vi "UHR-Fleezers Control (host) - 12.7d.vi"() -> ()   [LabVIEW 2012] (continued)
          }
          frame True {
            w4347 = TRUE ("AI to FIFO")
            n2449 = local read "Scan steps (MCL)"() -> (w4326:u64)
            n2450 = local read "Scan lines (y)"() -> (w4322:u64)
            n2451 = local read "Fast Scan Dir"() -> (w4333:bool)
            n2452 = local read "Actual MCL Inc (V)"() -> (w4323:dbl)
            n2453 = Decrement(x=w4322) -> (x-1=w4321:u64)
            n2454 = Decrement(x=w4326) -> (x-1=w4325:u64)
            n2455 = Multiply(x=w4323, y=w4321) -> (x*y=w4320:dbl)
            n2456 = Divide(x=w4320, y=2.0) -> (x/y=w4330:dbl)
            n2457 = Multiply(x=w4323, y=w4325) -> (x*y=w4324:dbl)
            n2458 = Divide(x=w4324, y=2.0) -> (x/y=w4329:dbl)
            n2459 = Select(t=w4329, s=w4333, f=w4330) -> (s? t:f=w4328:dbl)
            n2460 = Select(t=w4330, s=w4333, f=w4329) -> (s? t:f=w4332:dbl)
            n2461 = Subtract(x=w4340, y=w4332) -> (x-y=w4331:dbl)
            n2462 = Subtract(x=w4343, y=w4328) -> (x-y=w4327:dbl)
            n2463 = local read "2D or 1D Scan"() -> (w4345:bool)
            n2464 = Not(x=w4333) -> (.not. x?=w4339:bool)
            n2465 = Not(x=w4345) -> (.not. x?=w4341:bool)
            n2466 = And(x=w4333, y=w4341) -> (x .and. y?=w4342:bool)
            n2467 = And(x=w4341, y=w4339) -> (x .and. y?=w4344:bool)
            n2468 = Select(t=w4343, s=w4344, f=w4327) -> (s? t:f=w4334:dbl)
            n2469 = Select(t=w4340, s=w4342, f=w4331) -> (s? t:f=w4335:dbl)
            n2470 = call "Volt to I16.vi"("Voltage In"=w4335) -> ("I16 Voltage Out"=w4338:i16)
            n2471 = call "Volt to I16.vi"("Voltage In"=w4334) -> ("I16 Voltage Out"=w4337:i16)
            n2472 = xnode "Read/Write Control"("FPGA VI Reference In"=w4351, "error in"=w4350, "AI to FIFO"=w4347, "APD to FIFO"=w4347, "Start scan (MCL)"=w4347, "AO1"=w4338, "AO2"=w4337) -> ("FPGA VI Reference Out"=w4349:T20, "error out"=w4348:errorcluster)
          }
        }
        "Initial Y" <- w4300
        "Initial X" <- w4299
        n2473 = local write "Tab Control 6"(T3."Imaging" ("Tab Control 6")) -> ()
        "wait to reset values" <- w4301
      }
    }
    n2474 = local read "APD Elements/DMA read"() -> (w3455:u32)
    n2475 = local read "Trap AI Elements/DMA read"() -> (w3675:u32)
    n2476 = xnode "Get APD Data"("FPGA VI Reference In"=w3614, "error in"=w3613, "Number of Elements"=w3455, "Timeout (ms)"=-1) -> ("Data"=w3644:u32[], "Elements Remaining"=→"APD FIFO Elements Remaining":u32)  [unwired: 2 out]
    n2477 = local read "Trap Pos Elements/DMA read"() -> (w3610:u32)
    n2478 = xnode "Invoke Method"("FPGA VI Reference In"=w3614, "error in"=w3613, "Number of Elements"=w3610, "Timeout (ms)"=-1) -> ("Data"=w3574:u16[], "Elements Remaining"=→"Trap Pos FIFO El Remaining":u32)  [unwired: 2 out]
    n2479 = xnode "Get Trap Data"("FPGA VI Reference In"=w3614, "error in"=w3613, "Number of Elements"=w3675, "Timeout (ms)"=-1 ("Timeout")) -> ("FPGA VI Reference Out"=w3509:T20, "error out"=w3508:errorcluster, "Data"=w3575:i16[], "Elements Remaining"=w3797:u32)
    "FIFO El. Rem." <- w3797
    n2480 = local read "DMA Update Period (s)"() -> (w3676:dbl)
    n2481 = local read "Trap AI FIFO Depth"() -> (w3799:u32)
    n2482 = local read "Number of APDs"() -> (w3477:u8)
    n2483 = Decimate 1D Array(w3574) -> (w3571:u16[], w3573:u16[], w3572:u16[])
    n2484 = feedback #6(0.0) -> (w3603:dbl)
    n2485 = Add(x=w3676, y=w3603) -> (x+y=w3773:dbl)
    n2486 = feedback-in #6(w3773) -> ()
    n2487 = To Time Stamp(1:w3603) -> (0:w3602:timestamp)
    n2488 = Subtract(x=w3799, y=w3675) -> (x-y=w3798:u32)
    n2489 = To Unsigned Long Integer(number=w3571) -> (unsigned 32bit integer=w3570:u32[])
    n2490 = Join Numbers(hi=w3573, lo=w3572) -> ((hi.lo)=w3569:u32[])
    n2491 = Divide(x=w3797, y=w3798) -> (x/y=w3796:dbl)
    "Buffer Status" <- w3796
    n2492 = case "Deinterlace APD signals" shown="3, Default" w3477 {
      tunnel: [w3809 w3815] -> w3454
      tunnel: w3644 -> [w3810 w3814]
      tunnel: [w3808 w3813] -> w3453
      tunnel: [w3807 w3811] -> w3460
      frame 3, Default {
        n2493 = Decimate 1D Array "APD signals"(w3810) -> (w3809:u32[], w3808:u32[], w3807:u32[])
      }
      frame 2 {
        n2494 = Decimate 1D Array "APD signals"(w3814) -> (w3815:u32[], w3813:u32[])
        n2495 = Multiply(x=w3813, y=u32 0) -> (x*y=w3811:u32[])
      }
    }
    n2496 = Join Numbers(hi=w3570, lo=w3569) -> ((hi.lo)=w3563:u64[])
    n2497 = call "IR AOM word to freq - vec.vi"("Frequency Word In (double vec)"=w3563) -> ("Frequency Out"=w3609:dbl[])
    n2498 = Equal?(x=w3796, y=1.0) -> (x = y?=w3794:bool)
    n2499 = case "Alert buffer overflow" shown="True" w3794 {
      frame False {
      }
      frame True {
        n2500 = call <vilib>:"Beep.vi"() -> ()  [unwired: 3 in, 9 out]
        "Overflow (data lost)" <- TRUE ("Overflow (data lost)")
      }
    }
    n2501 = Decimate 1D Array(w3609) -> (w3608:dbl[], w3607:dbl[])
    n2502 = Build Array(w3608, w3607) -> (w3606:dbl[][])
    n2503 = Bundle(w3454, w3453, w3460) -> (w3458:cluster{u32[], u32[], u32[]})  [unwired: 1 in]
    n2504 = Build Array(w3454, w3453, w3460) -> (w3734:u32[][])
    n2505 = for {
      tunnel: w3454 -> [w3805] mode=indexing
      n2506 = call "Smart Buffer (DBL) 1.vi"("new element [write]"=w3805, "mode"=T21."write") -> ()  [unwired: 4 in, 6 out]
    }
    n2507 = local read "APD Integration Time (s)"() -> (w3470:dbl)
    n2508 = To Double Precision Float(number=w3734) -> (double precision float=w3735:dbl[][])
    n2509 = feedback #7 "APD3"(w3460) -> (w3476:u32[])
    n2510 = feedback #8 "APD2"(w3453) -> (w3632:u32[])
    n2511 = feedback #9 "APD1"(w3454) -> (w3733:u32[])
    n2512 = Build Array (concatenate)(w3632, w3453) -> (w3631:u32[])
    n2513 = Build Array (concatenate)(w3476, w3460) -> (w3475:u32[])
    n2514 = Build Array (concatenate)(w3733, w3454) -> (w3730:u32[])
    n2515 = for {
      tunnel: w3453 -> [w3804] mode=indexing
      n2516 = call "Smart Buffer (DBL) 2.vi"("new element [write]"=w3804, "mode"=T21."write") -> ()  [unwired: 4 in, 6 out]
    }
    n2517 = Array Size(array=w3730) -> (size(s)=w3727:i32)
    n2518 = Array Size(array=w3454) -> (size(s)=w3729:i32)
    n2519 = Multiply(x=w3729, y="APD Ave N") -> (x*y=w3728:dbl)
    n2520 = Greater?(x=w3727, y=w3728) -> (0:w3731:bool)
    n2521 = Bundle("APD 1", "APD 2", "APD 3") -> (w3767:cluster{string, string, string})  [unwired: 1 out]
    n2522 = local read "Trap Sets"() -> (w3674:u32)
    n2523 = case shown="True" w3731 {
      tunnel: w3730 -> [w4107 w4116]
      tunnel: [w4107 w4114] -> w3681
      tunnel: w3728 -> [_ w4109]
      tunnel: w3727 -> [_ w4115]
      tunnel: w3631 -> [w4106 w4113]
      tunnel: [w4106 w4112] -> w3629
      tunnel: w3475 -> [w4105 w4111]
      tunnel: [w4105 w4108] -> w3471
      frame False {
      }
      frame True {
        n2524 = Subtract(x=w4115, y=w4109) -> (x-y=w4110:dbl)
        n2525 = Array Subset "APD3"(array=w4111, index=w4110, length=w4109) -> (w4108:u32[])
        n2526 = Array Subset "APD2"(array=w4113, index=w4110, length=w4109) -> (w4112:u32[])
        n2527 = Array Subset "APD1"(array=w4116, index=w4110, length=w4109) -> (w4114:u32[])
      }
    }
    n2528 = feedback-in #7(w3471) -> ()
    n2529 = feedback-in #8(w3629) -> ()
    n2530 = feedback-in #9(w3681) -> ()
    n2531 = Cluster To Array(cluster=w3767) -> (array=w3764:string[])
    n2532 = for "APD" {
      tunnel: w3735 -> [w4363] mode=indexing
      tunnel: w3470 -> [w4370]
      tunnel: [w4366] -> w3633 mode=indexing
      tunnel: "APD Disp. Scale" -> [w4367]
      tunnel: w3764 -> [w4365] mode=indexing
      tunnel: "APD Disp. Downsample" -> [w4361]
      tunnel: [w4364] -> w3763
      workers-P: _ -> [_]
      tunnel: w3602 -> [w4360]
      n2533 = call "integrate 1D array interval - double.vi"("Ave N"=w4361, "Array In"=w4363) -> ("Array Out"=w4362:dbl[])  [unwired: 1 out]
      n2534 = Multiply(x=w4370, y=w4361) -> (x*y=w4364:dbl)
      n2535 = Divide(x=w4362, y=w4367) -> (x/y=w4368:dbl[])
      n2536 = Bundle By Name("t0"=w4360, "Y"=w4368, "dt"=w4364) -> (w4369:waveform(dbl))  [unwired: 1 out]
      n2537 = Set Waveform Attribute(5:w4365, 6:"NI_ChannelName" ("name"), 7:w4369) -> (3:w4366:waveform(dbl))  [unwired: 1 in, 2 out]
    }
    "APD Display Period (s)" <- w3763
    n2538 = Reciprocal(x=w3763) -> (1/x=→"APD Display Freq. (Hz)":dbl)
    n2539 = case "Deinterlace trap data, average down PSD" shown="2" w3674 {
      tunnel: w3575 -> [w4388 w4453]
      tunnel: [w4385 w4450] -> w3667
      tunnel: [w4388 w4452] -> w3566
      tunnel: "Detector Type" -> [w4387 w4448]
      tunnel: [w4386 w4451] -> w3666
      tunnel: [w4384 w4449] -> w3771
      frame 1, Default {
        n2540 = Divide(x=w4388, y=3276.7) -> (x/y=w4389:dbl[])
        n2541 = Decimate 1D Array(w4389) -> (w4398:dbl[], w4397:dbl[], w4396:dbl[], w4395:dbl[], w4394:dbl[], w4393:dbl[], w4392:dbl[], w4391:dbl[])
        n2542 = case shown="\"IR-QPD + PSD + FB-QPD position\"" w4387 {
          tunnel: w4398 -> [w4422 w4447]
          tunnel: w4397 -> [w4421 w4446]
          tunnel: w4396 -> [w4406 w4424]
          tunnel: w4395 -> [w4407 w4434]
          tunnel: w4394 -> [w4420 w4445]
          tunnel: w4393 -> [w4419 w4444]
          tunnel: w4392 -> [w4403 w4425]
          tunnel: w4391 -> [w4402 w4423]
          tunnel: [w4401 w4431] -> w4386
          tunnel: [w4400 w4430] -> w4385
          tunnel: [w4399 w4429] -> w4384
          frame "IR-QPD + PSD + FB-QPD", Default {
            w4399 = 0  # Channel pattern
            n2543 = Divide(x=w4422, y=w4407) -> (x/y=w4409:dbl[])
            n2544 = Divide(x=w4421, y=w4407) -> (x/y=w4408:dbl[])
            n2545 = Divide(x=w4420, y=w4403) -> (x/y=w4405:dbl[])
            n2546 = Divide(x=w4419, y=w4402) -> (x/y=w4404:dbl[])
            n2547 = Build Array(w4409, w4408, w4407, w4406, w4405, w4404, w4403, w4402) -> (w4400:dbl[][])
            n2548 = Bundle("T1 Y", "T1 X", "T1 Sum", "FB Sum", "PSD Y", "PSD X", "PSD Y Sum", "PSD X Sum") -> (w4418:T44)  [unwired: 1 out]
            n2549 = Cluster To Array(cluster=w4418) -> (array=w4401:string[])
          }
          frame "IR-QPD + PSD + FB-QPD position" {
            w4429 = 3  # Channel pattern
            n2550 = Negate(x=w4425) -> (-x=w4426:dbl[])
            n2551 = Divide(x=w4447, y=w4434) -> (x/y=w4436:dbl[])
            n2552 = Divide(x=w4446, y=w4434) -> (x/y=w4435:dbl[])
            n2553 = Divide(x=w4445, y=w4425) -> (x/y=w4433:dbl[])
            n2554 = Divide(x=w4444, y=w4426) -> (x/y=w4432:dbl[])
            n2555 = Build Array(w4436, w4435, w4434, w4423, w4424, w4433, w4432, w4425) -> (w4430:dbl[][])
            n2556 = Bundle("T1 Y", "T1 X", "T1 Sum", "FB X", "FB Sum", "PSD Y", "PSD X", "PSD Y Sum") -> (w4443:T44)  [unwired: 1 out]
            n2557 = Cluster To Array(cluster=w4443) -> (array=w4431:string[])
          }
        }
      }
      frame 2 {
        n2558 = case shown="\"IR-QPD + PSD + FB-QPD X position\"" w4448 {
          tunnel: w4453 -> [w4515 w4587 w4658]
          tunnel: [w4454 w4578 w4589] -> w4452
          tunnel: [w4481 w4569 w4636] -> w4451
          tunnel: [w4480 w4532 w4603] -> w4450
          tunnel: [w4474 w4567 w4634] -> w4449
          frame "IR-QPD + PSD + FB-QPD", Default {
            w4474 = 1  # Channel pattern
            # "time average x2 the 4th signal and the 4 psd signals (detection laser)"
            # "deinterlace 3 signals from qpd"
            n2559 = Decimate 1D Array(w4515) -> (w4514:i16[], w4513:i16[], w4479:i16[], w4512:i16[], w4502:i16[], w4500:i16[], w4499:i16[], w4497:i16[])
            n2560 = Decimate 1D Array(w4479) -> (w4478:i16[], w4477:i16[])
            n2561 = Decimate 1D Array(w4514) -> (w4511:i16[], w4483:i16[])
            n2562 = Decimate 1D Array(w4513) -> (w4510:i16[], w4508:i16[])
            n2563 = Decimate 1D Array(w4512) -> (w4509:i16[], w4507:i16[])
            n2564 = call "downsample 1D array - double.vi"("Ave N"=2.0, "Array In"=w4502) -> ("Array Out"=w4501:dbl[])  [unwired: 1 out]
            n2565 = call "downsample 1D array - double.vi"("Ave N"=2.0, "Array In"=w4500) -> ("Array Out"=w4482:dbl[])  [unwired: 1 out]
            n2566 = call "downsample 1D array - double.vi"("Ave N"=2.0, "Array In"=w4499) -> ("Array Out"=w4498:dbl[])  [unwired: 1 out]
            n2567 = call "downsample 1D array - double.vi"("Ave N"=2.0, "Array In"=w4497) -> ("Array Out"=w4496:dbl[])  [unwired: 1 out]
            n2568 = Interleave 1D Arrays(w4511, w4510, w4509, w4483, w4508, w4507, w4478, w4477, w4501, w4482, w4498, w4496) -> (w4495:dbl[])
            n2569 = Divide(x=w4495, y=3276.7) -> (x/y=w4494:dbl[])
            n2570 = Decimate 1D Array(w4494) -> (w4493:dbl[], w4492:dbl[], w4491:dbl[], w4490:dbl[], w4489:dbl[], w4488:dbl[], w4476:dbl[], w4475:dbl[], w4487:dbl[], w4486:dbl[], w4485:dbl[], w4484:dbl[])
            n2571 = Divide(x=w4493, y=w4491) -> (x/y=w4461:dbl[])
            n2572 = Divide(x=w4492, y=w4491) -> (x/y=w4460:dbl[])
            n2573 = Divide(x=w4490, y=w4488) -> (x/y=w4459:dbl[])
            n2574 = Divide(x=w4489, y=w4488) -> (x/y=w4458:dbl[])
            n2575 = Divide(x=w4487, y=w4485) -> (x/y=w4457:dbl[])
            n2576 = Divide(x=w4486, y=w4484) -> (x/y=w4456:dbl[])
            n2577 = Build Array(w4461, w4460, w4491, w4459, w4458, w4488, w4476, w4475, w4457, w4456, w4485, w4484) -> (w4480:dbl[][])
            n2578 = Bundle("T1 Y", "T1 X", "T1 Sum", "T2 Y", "T2 X", "T2 Sum", "T1 FB Sum", "T2 FB Sum", "PSD Y", "PSD X", "PSD Y Sum", "PSD X Sum") -> (w4462:T45)  [unwired: 1 out]
            n2579 = To Word Integer(number=w4495) -> (16bit integer=w4454:i16[])
            n2580 = Cluster To Array(cluster=w4462) -> (array=w4481:string[])
          }
          frame "IR-QPD + PSD + FB-QPD X position" {
            w4567 = 2  # Channel pattern
            # "time average x2 the 3 psd signals (detection laser)"
            # "deinterlace 3 signals from qpds"
            n2581 = Decimate 1D Array(w4587) -> (w4586:i16[], w4585:i16[], w4568:i16[], w4584:i16[], w4530:i16[], w4527:i16[], w4524:i16[], w4555:i16[])
            n2582 = Select(t=i16 -1, s="Flip X Sign", f=i16 1) -> (s? t:f=w4520:i16)
            n2583 = Multiply(x=w4585, y=w4520) -> (x*y=w4521:i16[])
            n2584 = Decimate 1D Array(w4568) -> (w4553:i16[], w4551:i16[])
            n2585 = Decimate 1D Array(w4586) -> (w4583:i16[], w4570:i16[])
            n2586 = Decimate 1D Array(w4521) -> (w4582:i16[], w4580:i16[])
            n2587 = Decimate 1D Array(w4584) -> (w4581:i16[], w4579:i16[])
            n2588 = Decimate 1D Array(w4555) -> (w4554:i16[], w4552:i16[])
            n2589 = call "downsample 1D array - I16.vi"("Ave N"=2.0, "Array In"=w4530) -> ("Array Out"=w4528:i16[])  [unwired: 1 in]
            n2590 = call "downsample 1D array - I16.vi"("Ave N"=2.0, "Array In"=w4524) -> ("Array Out"=w4522:i16[])  [unwired: 1 in]
            n2591 = call "downsample 1D array - I16.vi"("Ave N"=2.0, "Array In"=w4527) -> ("Array Out"=w4525:i16[])  [unwired: 1 in]
            n2592 = Interleave 1D Arrays(w4583, w4582, w4581, w4570, w4580, w4579, w4554, w4553, w4552, w4551, w4528, w4525, w4522) -> (w4578:i16[])
            n2593 = Divide(x=w4578, y=3276.7) -> (x/y=w4577:dbl[])
            n2594 = Decimate 1D Array(w4577) -> (w4576:dbl[], w4575:dbl[], w4574:dbl[], w4573:dbl[], w4572:dbl[], w4571:dbl[], w4543:dbl[], w4541:dbl[], w4540:dbl[], w4538:dbl[], w4537:dbl[], w4536:dbl[], w4533:dbl[])
            n2595 = Negate(x=w4533) -> (-x=w4531:dbl[])
            n2596 = Divide(x=w4537, y=w4533) -> (x/y=w4535:dbl[])
            n2597 = Divide(x=w4536, y=w4531) -> (x/y=w4534:dbl[])
            n2598 = Divide(x=w4576, y=w4574) -> (x/y=w4559:dbl[])
            n2599 = Divide(x=w4575, y=w4574) -> (x/y=w4558:dbl[])
            n2600 = Divide(x=w4573, y=w4571) -> (x/y=w4557:dbl[])
            n2601 = Divide(x=w4572, y=w4571) -> (x/y=w4556:dbl[])
            n2602 = Divide(x=w4543, y=w4541) -> (x/y=w4542:dbl[])
            n2603 = Divide(x=w4540, y=w4538) -> (x/y=w4539:dbl[])
            n2604 = Build Array(w4559, w4558, w4574, w4557, w4556, w4571, w4542, w4541, w4539, w4538, w4535, w4534, w4533) -> (w4532:dbl[][])
            n2605 = Bundle("T1 Y", "T1 X", "T1 Sum", "T2 Y", "T2 X", "T2 Sum", "T1 FB X", "T1 FB Sum", "T2 FB X", "T2 FB Sum", "PSD Y", "PSD X", "PSD Y Sum") -> (w4560:T46)  [unwired: 1 out]
            n2606 = Cluster To Array(cluster=w4560) -> (array=w4569:string[])
          }
          frame "IR-QPD + PSD + FB-QPD XY positions" {
            w4634 = 4  # Channel pattern
            # "time average x2 the 3 psd signals (detection laser)"
            # "deinterlace 3 signals from qpds"
            n2607 = Decimate 1D Array(w4658) -> (w4657:i16[], w4656:i16[], w4635:i16[], w4655:i16[], w4601:i16[], w4647:i16[], w4646:i16[], w4623:i16[])
            n2608 = Decimate 1D Array "Feedback Sum"(w4635) -> (w4619:i16[], w4617:i16[])
            n2609 = Decimate 1D Array "QPD Y"(w4657) -> (w4654:i16[], w4637:i16[])
            n2610 = Decimate 1D Array "QPD X"(w4656) -> (w4653:i16[], w4651:i16[])
            n2611 = Decimate 1D Array "Feedback Y"(w4601) -> (w4600:i16[], w4599:i16[])
            n2612 = Decimate 1D Array "QPD Sum"(w4655) -> (w4652:i16[], w4650:i16[])
            n2613 = Decimate 1D Array "Feedback X"(w4623) -> (w4620:i16[], w4618:i16[])
            n2614 = call "downsample 1D array - double.vi"("Ave N"=2.0, "Array In"=w4647) -> ("Array Out"=w4622:dbl[])  [unwired: 1 out]
            n2615 = call "downsample 1D array - double.vi"("Ave N"=2.0, "Array In"=w4646) -> ("Array Out"=w4621:dbl[])  [unwired: 1 out]
            n2616 = Interleave 1D Arrays(w4654, w4653, w4652, w4637, w4651, w4650, w4600, w4620, w4619, w4599, w4618, w4617, w4622, w4621) -> (w4645:dbl[])
            n2617 = Divide(x=w4645, y=3276.7) -> (x/y=w4644:dbl[])
            n2618 = Decimate 1D Array(w4644) -> (w4643:dbl[], w4642:dbl[], w4641:dbl[], w4640:dbl[], w4639:dbl[], w4638:dbl[], w4596:dbl[], w4610:dbl[], w4594:dbl[], w4595:dbl[], w4608:dbl[], w4592:dbl[], w4606:dbl[], w4604:dbl[])
            n2619 = Negate(x=w4604) -> (-x=w4602:dbl[])
            n2620 = Divide(x=w4606, y=w4602) -> (x/y=w4605:dbl[])
            n2621 = Divide(x=w4595, y=w4592) -> (x/y=w4591:dbl[])
            n2622 = Divide(x=w4596, y=w4594) -> (x/y=w4593:dbl[])
            n2623 = Divide(x=w4643, y=w4641) -> (x/y=w4627:dbl[])
            n2624 = Divide(x=w4642, y=w4641) -> (x/y=w4626:dbl[])
            n2625 = Divide(x=w4640, y=w4638) -> (x/y=w4625:dbl[])
            n2626 = Divide(x=w4639, y=w4638) -> (x/y=w4624:dbl[])
            n2627 = Divide(x=w4610, y=w4594) -> (x/y=w4609:dbl[])
            n2628 = Divide(x=w4608, y=w4592) -> (x/y=w4607:dbl[])
            n2629 = Build Array(w4627, w4626, w4641, w4625, w4624, w4638, w4593, w4609, w4594, w4591, w4607, w4592, w4605, w4604) -> (w4603:dbl[][])
            n2630 = Bundle("T1 Y", "T1 X", "T1 Sum", "T2 Y", "T2 X", "T2 Sum", "T1 FB Y", "T1 FB X", "T1 FB Sum", "T2 FB Y", "T2 FB X", "T2 FB Sum", "PSD X", "PSD Y Sum") -> (w4590:T47)  [unwired: 1 out]
            n2631 = To Word Integer(number=w4645) -> (16bit integer=w4589:i16[])
            n2632 = Cluster To Array(cluster=w4590) -> (array=w4636:string[])
          }
        }
      }
    }
    "AI labels" <- w3666
    n2633 = local read "APD Integration Time (s)"() -> (w3639:dbl)
    n2634 = Array Size(array=w3681) -> (size(s)=w3726:i32)
    n2635 = call <vilib>:"Std Deviation and Variance.vi"("X"=w3629) -> ("standard deviation"=w3628:dbl)  [unwired: 1 in, 2 out]
    n2636 = Add Array Elements(numeric array=w3629) -> (sum=w3630:u32)
    n2637 = Add Array Elements(numeric array=w3681) -> (sum=w3736:u32)
    n2638 = call <vilib>:"Std Deviation and Variance.vi"("X"=w3681) -> ("standard deviation"=w3680:dbl)  [unwired: 1 in, 2 out]
    n2639 = Divide(x=w3628, y=w3470) -> (x/y=w3625:dbl)
    "Rate sigma (Hz) 2" <- w3625
    n2640 = Multiply(x=w3470, y=w3726) -> (x*y=w3472:dbl)
    "Int. Time (s)" <- w3472
    n2641 = Divide(x=w3630, y=w3472) -> (x/y=w3626:dbl)
    "APD 2 Rate (Hz)" <- w3626
    n2642 = Multiply(x="APD Disp. Scale", y=w3633) -> (x*y=w3641:waveform(dbl)[])
    n2643 = Divide(x=w3736, y=w3472) -> (x/y=w3678:dbl)
    "APD 1 Rate (Hz)" <- w3678
    n2644 = Divide(x=w3680, y=w3470) -> (x/y=w3679:dbl)
    "Rate sigma (Hz)" <- w3679
    n2645 = Divide(x=w3625, y=w3626) -> (x/y=→"Sigma/Mean 2":dbl)
    n2646 = Multiply(x="APD Disp. Downsample", y=w3639) -> (x*y=w3637:dbl)
    n2647 = Divide(x=w3679, y=w3678) -> (x/y=→"Sigma/Mean":dbl)
    n2648 = Divide(x=w3641, y=w3637) -> (x/y=w3462:waveform(dbl)[])
    n2649 = Index Array(array=w3462, index=0) -> (element=w3622:waveform(dbl))
    n2650 = Index Array(array=w3462, index=1) -> (element=w3620:waveform(dbl))
    n2651 = Index Array(array=w3462, index=2) -> (element=w3464:waveform(dbl))
    n2652 = Subtract(x=w3622, y="APD 1 Offset") -> (x-y=w3618:waveform(dbl))
    n2653 = Subtract(x=w3620, y="APD 2 Offset") -> (x-y=w3617:waveform(dbl))
    n2654 = Subtract(x=w3464, y="APD 3 Offset") -> (x-y=w3461:waveform(dbl))
    n2655 = Add Array Elements(numeric array=w3471) -> (sum=w3474:u32)
    n2656 = call <vilib>:"Std Deviation and Variance.vi"("X"=w3471) -> ("standard deviation"=w3473:dbl)  [unwired: 1 in, 2 out]
    n2657 = Build Array(w3618, w3617, w3461) -> (→"APD Chart":waveform(dbl)[])
    n2658 = Divide(x=w3474, y=w3472) -> (x/y=w3468:dbl)
    "APD 3 Rate (Hz)" <- w3468
    n2659 = Divide(x=w3473, y=w3470) -> (x/y=w3469:dbl)
    "Rate sigma (Hz) 3" <- w3469
    n2660 = Divide(x=w3469, y=w3468) -> (x/y=→"Sigma/Mean 3":dbl)
    n2661 = local read "Data Period (s)"() -> (w3525:dbl)
    n2662 = local read "BD 1 Frequency 2 (MHz)"() -> (w3558:dbl)
    n2663 = local read "BD 1 Frequency 1 (MHz)"() -> (w3559:dbl)
    n2664 = Decimate 1D Array(w3566) -> (w3590:i16[], w3589:i16[], w3587:i16[], w3586:i16[])  [unwired: 9 out]
    n2665 = Multiply(x=w3525, y="Trap Pos. Disp. Downsample") -> (x*y=w3523:dbl)
    n2666 = Divide(x=w3590, y=w3589) -> (x/y=w3591:dbl[])
    n2667 = Divide(x=w3587, y=w3586) -> (x/y=w3588:dbl[])
    n2668 = local read "AOM X Cal (nm/MHz)"() -> (w3556:dbl)
    n2669 = Split 1D Array(array=w3591, index="N El. to Ave.") -> (second subarray=w3594:dbl[])  [unwired: 1 out]
    n2670 = Split 1D Array(array=w3588, index="N El. to Ave.") -> (second subarray=w3593:dbl[])  [unwired: 1 out]
    n2671 = Multiply(x=w3525, y="Trap Disp. Downsample") -> (x*y=w3604:dbl)
    "Display Period (s)" <- w3604
    n2672 = for "Trap AI" {
      tunnel: [w4383] -> w3447 mode=indexing
      tunnel: w3602 -> [w4374]
      tunnel: "Trap Disp. Downsample" -> [w4381]
      tunnel: w3667 -> [w4379] mode=indexing
      tunnel: w3525 -> [w4378]
      tunnel: w3666 -> [w4377] mode=indexing
      tunnel: [w4376] -> w3636 mode=indexing
      tunnel: w3604 -> [w4375]
      workers-P: _ -> [_]
      n2673 = Bundle By Name("Y"=w4379, "dt"=w4378) -> (w4380:waveform(dbl))  [unwired: 1 out]
      n2674 = Set Waveform Attribute(5:w4377, 6:"NI_ChannelName" ("name"), 7:w4380) -> (3:w4376:waveform(dbl))  [unwired: 1 in, 2 out]
      n2675 = call "downsample 1D array - double.vi"("Ave N"=w4381, "Array In"=w4379) -> ("Array Out"=w4382:dbl[])  [unwired: 1 out]
      n2676 = Bundle By Name(cluster=w4376, "t0"=w4374, "Y"=w4382, "dt"=w4375) -> (w4383:waveform(dbl))
    }
    n2677 = Bundle("BD 1 Frequency 1 (MHz)"=w3559, "BD 1 Frequency 2 (MHz)"=w3558) -> (w3560:T48)  [unwired: 1 out]
    n2678 = call-poly <vilib>:"Mean.vi"("X"=w3593) -> ("mean"=w3581:dbl)  [unwired: 1 out]
    n2679 = call-poly <vilib>:"Mean.vi"("X"=w3594) -> ("mean"=w3582:dbl)  [unwired: 1 out]
    n2680 = Reciprocal(x=w3604) -> (1/x=→"Trap Disp. Freq. (Hz)":dbl)
    n2681 = Cluster To Array(cluster=w3560) -> (array=w3557:dbl[])
    n2682 = local read "Trap X AI1 (DMA)"() -> (w3592:T13)
    n2683 = local read "Data points/scans (MCL)"() -> (w3746:dbl)
    n2684 = To Fixed-Point(number=w3581) -> (fixed-point=w3579:fxp<+/-,16,1>)  [unwired: 1 in]
    n2685 = To Fixed-Point(number=w3582) -> (fixed-point=w3580:fxp<+/-,16,1>)  [unwired: 1 in]
    n2686 = Bundle("Trap 1 Pos.", "Trap 2 Pos.") -> (w3601:cluster{string, string})  [unwired: 1 out]
    n2687 = Bundle By Name(cluster=w3592, "Set 1"=w3580, "Set 2"=w3579) -> (→"Trap X AI1 (DMA)":T13)
    n2688 = Cluster To Array(cluster=w3601) -> (array=w3598:string[])
    n2689 = Unbundle(w3458) -> (w3459:u32[])  [unwired: 2 out]
    n2690 = Select(t=-1.0, s="Negate Y Axis", f=1.0) -> (s? t:f=w3542:dbl)
    n2691 = for "Trap Position" {
      tunnel: w3606 -> [w3975] mode=indexing
      tunnel: "Trap Pos. Disp. Downsample" -> [w3974]
      tunnel: w3523 -> [w3972]
      tunnel: w3602 -> [w3971]
      tunnel: w3598 -> [w3969] mode=indexing
      tunnel: [w3968] -> w3512 mode=indexing
      tunnel: w3557 -> [w3966] mode=indexing
      tunnel: w3556 -> [w3964]
      tunnel: w3542 -> [w3963]
      n2692 = call "downsample 1D array - double.vi"("Ave N"=w3974, "Array In"=w3975) -> ("Array Out"=w3973:dbl[])  [unwired: 1 out]
      n2693 = Subtract(x=w3973, y=w3966) -> (x-y=w3967:dbl[])
      n2694 = Multiply(x=w3964, y=w3967) -> (x*y=w3965:dbl[])
      n2695 = Multiply(x=w3963, y=w3965) -> (x*y=w3962:dbl[])
      n2696 = Bundle By Name("Y"=w3962, "dt"=w3972, "t0"=w3971) -> (w3970:waveform(dbl))  [unwired: 1 out]
      n2697 = Set Waveform Attribute(5:w3969, 6:"NI_ChannelName" ("name"), 7:w3970) -> (3:w3968:waveform(dbl))  [unwired: 1 in, 2 out]
    }
    n2698 = To Double Precision Float(number=w3459) -> (double precision float=w3664:dbl[])
    n2699 = local read "Display Period (s)"() -> (w3653:dbl)
    n2700 = Increment(x=w3746) -> (x+1=w3747:dbl)
    n2701 = Index Array(array=w3512, index=0) -> (element=w3516:waveform(dbl))
    n2702 = Index Array(array=w3512, index=1) -> (element=w3511:waveform(dbl))
    n2703 = feedback #10(w3747) -> (w3750:dbl)
    n2704 = Select(t=0, s=w3737, f=w3750) -> (s? t:f=w3743:dbl)
    n2705 = Array Size(array=w3664) -> (size(s)=w3749:i32)
    n2706 = Build Array (concatenate)(w3633, w3447) -> (w3452:waveform(dbl)[])
    "All Signals" <- w3452
    n2707 = Add(x=w3749, y=w3743) -> (x+y=w3744:dbl)
    n2708 = Unbundle By Name(w3516) -> ("Y"=w3517:dbl[])
    n2709 = Divide(x="Bead Sep. Int. Time (s)", y=w3653) -> (x/y=w3552:dbl)
    n2710 = Add(x=w3517, y="FB Trap Pos Offset") -> (x+y=w3515:dbl[])
    "T1 x pos data" <- w3515
    n2711 = Greater?(x=w3744, y=w3746) -> (0:w3745:bool)
    n2712 = feedback #11(w3515) -> (w3554:dbl[])
    n2713 = Build Array (concatenate)(w3515, w3554) -> (w3553:dbl[])
    n2714 = Bundle By Name(cluster=w3516, "Y"=w3515) -> (w3514:waveform(dbl))
    n2715 = Select(t=w3743, s=w3745, f=w3744) -> (s? t:f=w3742:dbl)
    n2716 = feedback-in #10(w3742) -> ()
    n2717 = local read "MCL Scanning"() -> (w3740:bool)
    n2718 = Bundle(w3514, w3511) -> (w3510:cluster{waveform(dbl), waveform(dbl)})  [unwired: 1 out]
    n2719 = Index Array(array=w3447, index="index 1") -> (element=w3446:waveform(dbl))
    n2720 = Index Array(array=w3447, index="index 2") -> (element=w3451:waveform(dbl))
    n2721 = Split 1D Array(array=w3553, index=w3552) -> (first subarray=w3546:dbl[])  [unwired: 1 out]
    n2722 = feedback-in #11(w3546) -> ()
    n2723 = Unbundle By Name(w3446) -> ("Y"=w3445:dbl[])
    n2724 = Unbundle By Name(w3451) -> ("Y"=w3450:dbl[])
    n2725 = Not(x=w3745) -> (.not. x?=w3739:bool)
    n2726 = Cluster To Array(cluster=w3510) -> (array=w3486:waveform(dbl)[])
    "Trap Positions" <- w3486
    n2727 = call-poly <vilib>:"Mean.vi"("X"=w3546) -> ("mean"=w3545:dbl)  [unwired: 1 out]
    "Mean T1 Position (nm)" <- w3545
    n2728 = Subtract(x=w3546, y=w3545) -> (x-y=w3551:dbl[])
    n2729 = Square(x=w3551) -> (x^2=w3550:dbl[])
    n2730 = And(x=w3739, y=w3740) -> (x .and. y?=w3741:bool)
    n2731 = call-poly <vilib>:"Mean.vi"("X"=w3550) -> ("mean"=w3549:dbl)  [unwired: 1 out]
    n2732 = call-poly <vilib>:"Mean.vi"("X"=w3445) -> ("mean"=→"Trap 1 sum mean":dbl)  [unwired: 1 out]
    n2733 = call-poly <vilib>:"Mean.vi"("X"=w3450) -> ("mean"=→"Trap 2 sum mean":dbl)  [unwired: 1 out]
    n2734 = Square Root(x=w3549) -> (sqrt(x)=w3548:dbl)
    n2735 = Or(x=w3741, y=w3737) -> (x .or. y?=w3738:bool)
    n2736 = Equal?(x="Tab Control 6", y=T38."High Res Display") -> (x = y?=w3670:bool)
    n2737 = Multiply(x=10.0, y=w3548) -> (x*y=→"Trap 1 Position RMS (A)":dbl)
    n2738 = case "For displaying the high resolution display (no downsampling)" shown="True" w3670 {
      tunnel: w3636 -> [_ w3995]
      frame False {
      }
      frame True {
        n2739 = Index Array(array=w3995, index="High Res. Display") -> (element=w3996:waveform(dbl))
        n2740 = call <vilib>:"Std Deviation and Variance.vi"("X"=w3996) -> ("mean"=w4003:dbl, "standard deviation"=w4008:dbl)  [unwired: 1 in, 1 out]
        "Mean Intensity" <- w4003
        "Sigma" <- w4008
        n2741 = Subtract(x=w3996, y=w4003) -> (x-y=w4002:waveform(dbl))
        n2742 = Select(t=w4002, s="Subtract mean", f=w3996) -> (s? t:f=→"1 Channel":waveform(dbl))
        n2743 = Divide(x=w4008, y=w4003) -> (x/y=→"Sigma/Mean":dbl)
        n2744 = feedback #12(1) -> (w3997:i32)
        n2745 = Greater Or Equal?(x=w3997, y="Slow mean N ave.") -> (x >= y?=w4010:bool)
        n2746 = Increment(x=w3997) -> (x+1=w4012:i32)
        n2747 = Select(t=1, s=w4010, f=w4012) -> (s? t:f=w3999:i32)
        n2748 = feedback-in #12(w3999) -> ()
        n2749 = feedback #13() -> (w4000:waveform(dbl))  [unwired: 1 out]
        n2750 = case shown="Default" w3997 {
          tunnel: [w4015 w4018] -> w4001
          tunnel: w4000 -> [w4017 _]
          tunnel: w3996 -> [w4016 w4018]
          frame Default {
            n2751 = call-poly <vilib>:"Append Waveforms.vi"("waveform B"=w4016, "waveform A"=w4017) -> ("waveform out"=w4015:waveform(dbl))  [unwired: 1 in, 8 out]
          }
          frame 1 {
          }
        }
        n2752 = feedback-in #13(w4001) -> ()
        n2753 = case shown="True" w4010 {
          tunnel: w4001 -> [_ w4014]
          frame False {
          }
          frame True {
            n2754 = call-poly <vilib>:"Mean.vi"("X"=w4014) -> ("mean"=→"Slow mean":dbl)  [unwired: 1 out]
          }
        }
      }
    }
    n2755 = case "For plotting results of scanning MCL (fluorescence and detection laser images)" shown="True" w3738 {
      tunnel: w3737 -> [_ w4122]
      tunnel: w3746 -> [_ _]
      tunnel: w3636 -> [_ w4251]
      tunnel: w3615 -> [_ w4159]
      tunnel: w3458 -> [_ w4129]
      frame False {
      }
      frame True {
        w4139 = u32 0 items=["Horizontal", "Vertical", "Central", "1st Diagonal", "2nd Diagonal"] ("Type of Symmetry")
        w4166 = u32 0 items=["Horizontal", "Vertical", "Central", "1st Diagonal", "2nd Diagonal"] ("Type of Symmetry")
        w4190 = u32 0 items=["Horizontal", "Vertical", "Central", "1st Diagonal", "2nd Diagonal"] ("Type of Symmetry")
        w4193 = u32 0 items=["Horizontal", "Vertical", "Central", "1st Diagonal", "2nd Diagonal"] ("Type of Symmetry")
        w4222 = u32 0 items=["Horizontal", "Vertical", "Central", "1st Diagonal", "2nd Diagonal"] ("Type of Symmetry")
        n2756 = Unbundle(w4129) -> (w4128:u32[], w4126:u32[], w4124:u32[])
        n2757 = To Double Precision Float(number=w4128) -> (double precision float=w4127:dbl[])
        n2758 = To Double Precision Float(number=w4126) -> (double precision float=w4125:dbl[])
        n2759 = To Double Precision Float(number=w4124) -> (double precision float=w4123:dbl[])
        n2760 = Index Array(array=w4251, index=10) -> (element=w4257:waveform(dbl))
        n2761 = Index Array(array=w4251, index=11) -> (element=w4254:waveform(dbl))
        n2762 = local read "Cycles/step (MCL)"() -> (w4207:u64)
        n2763 = Index Array(array=w4251, index="Channel") -> (element=w4253:waveform(dbl))
        n2764 = Unbundle(w4159) -> ("New Image"=w4158:T2, "New Image"=w4157:T2, "New Image"=w4130:T2, "New Image"=w4131:T2, "New Image"=w4132:T2)
        n2765 = local read "Scan steps (MCL)"() -> (w4118:u64)
        n2766 = Unbundle By Name(w4257) -> ("Y"=w4209:dbl[])
        n2767 = Unbundle By Name(w4254) -> ("Y"=w4211:dbl[])
        n2768 = local read "Scan lines (y)"() -> (w4119:u64)
        n2769 = local read "N APD Samp/step"() -> (w4121:dbl)
        n2770 = Unbundle By Name(w4253) -> ("Y"=w4216:dbl[])
        n2771 = call "downsample 1D array - double.vi"("Ave N"=w4207, "Array In"=w4209) -> ("Array Out"=w4208:dbl[])  [unwired: 1 out]
        n2772 = call "downsample 1D array - double.vi"("Ave N"=w4207, "Array In"=w4211) -> ("Array Out"=w4210:dbl[])  [unwired: 1 out]
        n2773 = call "downsample 1D array - double.vi"("Ave N"=w4207, "Array In"=w4216) -> ("Array Out"=w4215:dbl[])  [unwired: 1 out]
        n2774 = Multiply(x=w4118, y=u64 2) -> (x*y=w4120:u64)
        n2775 = feedback #14(w4125) -> (w4184:dbl[])
        n2776 = Build Array (concatenate)(w4184, w4125) -> (w4183:dbl[])
        n2777 = feedback #15(w4123) -> (w4156:dbl[])
        n2778 = Build Array (concatenate)(w4156, w4123) -> (w4117:dbl[])
        n2779 = Select(t=w4125, s=w4122, f=w4183) -> (s? t:f=w4168:dbl[])
        n2780 = feedback-in #14(w4168) -> ()
        n2781 = Select(t=w4123, s=w4122, f=w4117) -> (s? t:f=w4141:dbl[])
        n2782 = feedback-in #15(w4141) -> ()
        n2783 = feedback #16(w4127) -> (w4277:dbl[])
        n2784 = Build Array (concatenate)(w4277, w4127) -> (w4259:dbl[])
        n2785 = Select(t=w4127, s=w4122, f=w4259) -> (s? t:f=w4263:dbl[])
        n2786 = feedback-in #16(w4263) -> ()
        n2787 = feedback #17(w4208) -> (w4265:dbl[])
        n2788 = Build Array (concatenate)(w4265, w4208) -> (w4256:dbl[])
        n2789 = feedback #18(w4215) -> (w4275:dbl[])
        n2790 = Build Array (concatenate)(w4275, w4215) -> (w4274:dbl[])
        n2791 = feedback #19(w4210) -> (w4267:dbl[])
        n2792 = Build Array (concatenate)(w4267, w4210) -> (w4268:dbl[])
        n2793 = Select(t=w4208, s=w4122, f=w4256) -> (s? t:f=w4212:dbl[])
        n2794 = feedback-in #17(w4212) -> ()
        n2795 = Select(t=w4215, s=w4122, f=w4274) -> (s? t:f=w4214:dbl[])
        n2796 = feedback-in #18(w4214) -> ()
        n2797 = Select(t=w4210, s=w4122, f=w4268) -> (s? t:f=w4213:dbl[])
        n2798 = feedback-in #19(w4213) -> ()
        n2799 = call "integrate 1D array interval - double.vi"("Ave N"=w4121, "Array In"=w4168) -> ("Array Out"=w4179:dbl[])  [unwired: 1 out]
        n2800 = call "integrate 1D array interval - double.vi"("Ave N"=w4121, "Array In"=w4141) -> ("Array Out"=w4152:dbl[])  [unwired: 1 out]
        n2801 = call "integrate 1D array interval - double.vi"("Ave N"=w4121, "Array In"=w4263) -> ("Array Out"=w4262:dbl[])  [unwired: 1 out]
        n2802 = Array Size(array=w4179) -> (size(s)=w4180:i32)
        n2803 = Array Size(array=w4152) -> (size(s)=w4153:i32)
        n2804 = Array Size(array=w4262) -> (size(s)=w4264:i32)
        n2805 = Multiply(x=w4119, y=w4120) -> (x*y=w4182:u64)
        n2806 = Multiply(x=w4119, y=w4120) -> (x*y=w4155:u64)
        n2807 = Multiply(x=w4119, y=w4120) -> (x*y=w4272:u64)
        n2808 = Subtract(x=w4182, y=w4180) -> (x-y=w4173:u64)
        n2809 = call-poly <vilib>:"Mean.vi"("X"=w4179) -> ("mean"=w4170:dbl)  [unwired: 1 out]
        n2810 = Subtract(x=w4155, y=w4153) -> (x-y=w4146:u64)
        n2811 = call-poly <vilib>:"Mean.vi"("X"=w4152) -> ("mean"=w4143:dbl)  [unwired: 1 out]
        n2812 = Subtract(x=w4272, y=w4264) -> (x-y=w4206:u64)
        n2813 = call-poly <vilib>:"Mean.vi"("X"=w4262) -> ("mean"=w4203:dbl)  [unwired: 1 out]
        n2814 = call-poly <vilib>:"Mean.vi"("X"=w4212) -> ("mean"=w4196:dbl)  [unwired: 1 out]
        n2815 = call-poly <vilib>:"Mean.vi"("X"=w4214) -> ("mean"=w4201:dbl)  [unwired: 1 out]
        n2816 = call-poly <vilib>:"Mean.vi"("X"=w4213) -> ("mean"=w4199:dbl)  [unwired: 1 out]
        n2817 = Initialize Array(1.0 ("element"), w4173) -> (w4169:dbl[])
        n2818 = Initialize Array(1.0 ("element"), w4146) -> (w4142:dbl[])
        n2819 = Initialize Array(1.0 ("element"), w4206) -> (w4197:dbl[])
        n2820 = Multiply(x=w4169, y=w4170) -> (x*y=w4171:dbl[])
        n2821 = Multiply(x=w4142, y=w4143) -> (x*y=w4144:dbl[])
        n2822 = Multiply(x=w4197, y=w4203) -> (x*y=w4204:dbl[])
        n2823 = Multiply(x=w4197, y=w4199) -> (x*y=w4200:dbl[])
        n2824 = Multiply(x=w4197, y=w4201) -> (x*y=w4202:dbl[])
        n2825 = Multiply(x=w4197, y=w4196) -> (x*y=w4198:dbl[])
        n2826 = Build Array (concatenate)(w4179, w4171) -> (w4181:dbl[])
        n2827 = Build Array (concatenate)(w4152, w4144) -> (w4154:dbl[])
        n2828 = Build Array (concatenate)(w4262, w4204) -> (w4271:dbl[])
        n2829 = Build Array (concatenate)(w4212, w4198) -> (w4266:dbl[])
        n2830 = Build Array (concatenate)(w4214, w4202) -> (w4270:dbl[])
        n2831 = Build Array (concatenate)(w4213, w4200) -> (w4269:dbl[])
        n2832 = Reshape Array(w4181, w4119, w4120) -> (w4177:dbl[][])
        n2833 = Reshape Array(w4154, w4119, w4120) -> (w4150:dbl[][])
        n2834 = Reshape Array(w4271, w4119, w4120) -> (w4249:dbl[][])
        n2835 = Reshape Array(w4266, w4119, w4120) -> (w4232:dbl[][])
        n2836 = Reshape Array(w4270, w4119, w4120) -> (w4224:dbl[][])
        n2837 = Reshape Array(w4269, w4119, w4120) -> (w4239:dbl[][])
        n2838 = Array Subset(array=w4177, index (col)=0 ("index"), length (col)=w4118) -> (w4176:dbl[][])  [unwired: 2 in]
        n2839 = Array Subset(array=w4177, index (col)=w4118) -> (w4174:dbl[][])  [unwired: 3 in]
        n2840 = Array Subset(array=w4150, index (col)=0 ("index"), length (col)=w4118) -> (w4149:dbl[][])  [unwired: 2 in]
        n2841 = Array Subset(array=w4150, index (col)=w4118) -> (w4147:dbl[][])  [unwired: 3 in]
        n2842 = Array Subset(array=w4239, index (col)=0 ("index"), length (col)=w4118) -> (w4244:dbl[][])  [unwired: 2 in]
        n2843 = Array Subset(array=w4239, index (col)=w4118) -> (w4242:dbl[][])  [unwired: 3 in]
        n2844 = Array Subset(array=w4249, index (col)=0 ("index"), length (col)=w4118) -> (w4248:dbl[][])  [unwired: 2 in]
        n2845 = Array Subset(array=w4249, index (col)=w4118) -> (w4246:dbl[][])  [unwired: 3 in]
        n2846 = Array Subset(array=w4224, index (col)=0 ("index"), length (col)=w4118) -> (w4230:dbl[][])  [unwired: 2 in]
        n2847 = Array Subset(array=w4224, index (col)=w4118) -> (w4228:dbl[][])  [unwired: 3 in]
        n2848 = Array Subset(array=w4232, index (col)=0 ("index"), length (col)=w4118) -> (w4237:dbl[][])  [unwired: 2 in]
        n2849 = Array Subset(array=w4232, index (col)=w4118) -> (w4235:dbl[][])  [unwired: 3 in]
        n2850 = for {
          tunnel: w4176 -> [w4281] mode=indexing
          tunnel: [w4280] -> w4175 mode=indexing
          workers-P: _ -> [_]
          n2851 = Reverse 1D Array(array=w4281) -> (reversed array=w4280:dbl[])
        }
        n2852 = for {
          tunnel: w4149 -> [w4279] mode=indexing
          tunnel: [w4278] -> w4148 mode=indexing
          workers-P: _ -> [_]
          n2853 = Reverse 1D Array(array=w4279) -> (reversed array=w4278:dbl[])
        }
        n2854 = for {
          tunnel: w4244 -> [w4287] mode=indexing
          tunnel: [w4286] -> w4243 mode=indexing
          workers-P: _ -> [_]
          n2855 = Reverse 1D Array(array=w4287) -> (reversed array=w4286:dbl[])
        }
        n2856 = for {
          tunnel: w4248 -> [w4289] mode=indexing
          tunnel: [w4288] -> w4247 mode=indexing
          workers-P: _ -> [_]
          n2857 = Reverse 1D Array(array=w4289) -> (reversed array=w4288:dbl[])
        }
        n2858 = for {
          tunnel: w4230 -> [w4283] mode=indexing
          tunnel: [w4282] -> w4229 mode=indexing
          workers-P: _ -> [_]
          n2859 = Reverse 1D Array(array=w4283) -> (reversed array=w4282:dbl[])
        }
        n2860 = for {
          tunnel: w4237 -> [w4285] mode=indexing
          tunnel: [w4284] -> w4236 mode=indexing
          workers-P: _ -> [_]
          n2861 = Reverse 1D Array(array=w4285) -> (reversed array=w4284:dbl[])
        }
        n2862 = Index Array(array=w4249, index (row)=0) -> (element=→"Waveform Graph":dbl[])  [unwired: 1 in]
        n2863 = Add(x=w4175, y=w4174) -> (x+y=w4161:dbl[][])
        n2864 = Add(x=w4148, y=w4147) -> (x+y=w4134:dbl[][])
        n2865 = Add(x=w4243, y=w4242) -> (x+y=w4241:dbl[][])
        n2866 = Add(x=w4247, y=w4246) -> (x+y=w4221:dbl[][])
        n2867 = Add(x=w4229, y=w4228) -> (x+y=w4227:dbl[][])
        n2868 = Add(x=w4236, y=w4235) -> (x+y=w4234:dbl[][])
        n2869 = Divide(x=w4227, y=2) -> (x/y=w4225:dbl[][])
        n2870 = Divide(x=w4241, y=2) -> (x/y=w4186:dbl[][])
        n2871 = To Single Precision Float(number=w4221) -> (single precision float=w4220:sgl[][])
        n2872 = To Single Precision Float(number=w4161) -> (single precision float=w4165:sgl[][])
        n2873 = To Single Precision Float(number=w4134) -> (single precision float=w4138:sgl[][])
        n2874 = Divide(x=w4234, y=2) -> (x/y=w4188:dbl[][])
        n2875 = Transpose 2D Array(2D array=w4225) -> (transposed array=→"Data map":dbl[][])
        n2876 = To Single Precision Float(number=w4186) -> (single precision float=w4192:sgl[][])
        n2877 = To Single Precision Float(number=w4188) -> (single precision float=w4189:sgl[][])
        n2878 = call "IMAQ ArrayToImage"("Image Pixels (Float)"=w4220, "Image"=w4158) -> ("Image Out"=w4223:T2)  [unwired: 8 in, 1 out]
        n2879 = call "IMAQ ArrayToImage"("Image Pixels (Float)"=w4165, "Image"=w4157) -> ("Image Out"=w4167:T2)  [unwired: 8 in, 1 out]
        n2880 = call "IMAQ ArrayToImage"("Image Pixels (Float)"=w4138, "Image"=w4130) -> ("Image Out"=w4140:T2)  [unwired: 8 in, 1 out]
        n2881 = call "IMAQ ArrayToImage"("Image Pixels (Float)"=w4192, "Image"=w4131) -> ("Image Out"=w4194:T2)  [unwired: 8 in, 1 out]
        n2882 = call "IMAQ Symmetry"("Type of Symmetry"=w4222, "Image Src"=w4223) -> ("Image Dst Out"=w4218:T2)  [unwired: 3 in, 1 out]
        n2883 = call "IMAQ ArrayToImage"("Image Pixels (Float)"=w4189, "Image"=w4132) -> ("Image Out"=w4191:T2)  [unwired: 8 in, 1 out]
        n2884 = call "IMAQ Symmetry"("Type of Symmetry"=w4166, "Image Src"=w4167) -> ("Image Dst Out"=w4163:T2)  [unwired: 3 in, 1 out]
        n2885 = call "IMAQ Symmetry"("Type of Symmetry"=w4139, "Image Src"=w4140) -> ("Image Dst Out"=w4136:T2)  [unwired: 3 in, 1 out]
        n2886 = call "IMAQ Symmetry"("Type of Symmetry"=w4193, "Image Src"=w4194) -> ("Image Dst Out"=→"Detection Laser X":T2)  [unwired: 3 in, 1 out]
        n2887 = call "IMAQ Symmetry"("Type of Symmetry"=w4190, "Image Src"=w4191) -> ("Image Dst Out"=→"Detection Laser Y":T2)  [unwired: 3 in, 1 out]
        n2888 = call "IMAQ Set Simple Calibration"("Calibration Axis Info"=T39 {"Origin Pixel"={"X"=0.0, "Y"=0.0}, "Angle Relative to Horizontal (deg)"=0.0, "Axis Reference"=0}, "Grid Descriptor"=T40 {"X Step"=0.3, "Y Step"=0.3, "Unit"=enum."Undefined"}, "Image"=w4218) -> ("Calibrated Image"=→"APD 1":T2)  [unwired: 7 in, 1 out]
        n2889 = call "IMAQ Set Simple Calibration"("Calibration Axis Info"=T39 {"Origin Pixel"={"X"=0.0, "Y"=0.0}, "Angle Relative to Horizontal (deg)"=0.0, "Axis Reference"=0}, "Grid Descriptor"=T40 {"X Step"=0.3, "Y Step"=0.3, "Unit"=enum."Undefined"}, "Image"=w4163) -> ("Calibrated Image"=→"APD 2":T2)  [unwired: 7 in, 1 out]
        n2890 = call "IMAQ Set Simple Calibration"("Calibration Axis Info"=T39 {"Origin Pixel"={"X"=0.0, "Y"=0.0}, "Angle Relative to Horizontal (deg)"=0.0, "Axis Reference"=0}, "Grid Descriptor"=T40 {"X Step"=0.3, "Y Step"=0.3, "Unit"=enum."Undefined"}, "Image"=w4136) -> ("Calibrated Image"=→"APD 3":T2)  [unwired: 7 in, 1 out]
      }
    }
    n2891 = case "For computing FFTs for display" shown="True" "Compute FFT" {
      tunnel: w3636 -> [_ w4761]
      frame False {
      }
      frame True {
        n2892 = Build Array("FFT 1 Choice 1", "FFT 1 Choice 2", "FFT 2 Choice 1", "FFT 2 Choice 2") -> (w4754:u16[])
        n2893 = Array Size(array=w4761) -> (size(s)=w4760:i32)
        n2894 = feedback-in #20(w4754) -> ()
        n2895 = feedback #20(u16[] [100, 100, 100, 100]) -> (w4755:u16[])
        n2896 = feedback-in #21("# Spectra to Ave.") -> ()
        n2897 = feedback #21("# Spectra to Ave.") -> (w4752:dbl)
        n2898 = Not Equal?(x="# Spectra to Ave.", y=w4752) -> (x != y?=w4751:bool)
        n2899 = Not Equal?(x=w4754, y=w4755) -> (x != y?=w4753:bool)
        n2900 = feedback #22(1.0) -> (w4738:dbl)
        n2901 = Compound Arithmetic op=OR("Reset FFT", w4753, w4751) -> (w4736:bool)
        n2902 = Select(t=1.0, s=w4736, f=w4738) -> (s? t:f=w4740:dbl)
        n2903 = Greater?(x=w4740, y="# Spectra to Ave.") -> (0:w4759:bool)
        n2904 = Increment(x=w4740) -> (x+1=w4739:dbl)
        n2905 = feedback-in #22(w4739) -> ()
        n2906 = local read "DMA Update Period (s)"() -> (w4734:dbl)
        n2907 = Multiply(x="# Spectra to Ave.", y=w4734) -> (x*y=→"Ave. Time (s)":dbl)
        n2908 = Build Array(cluster{"f0":dbl, "df":dbl, "magnitude":dbl[]} {"f0"=0.0, "df"=0.0, "magnitude"=[]} ("PSD")) -> (w4743:cluster{"f0":dbl, "df":dbl, "magnitude":dbl[]}[])
        n2909 = Build Array(w4743, w4743, w4743, w4743) -> (w4745:T49)
        n2910 = feedback #23(w4745) -> (w4750:T49)
        n2911 = for {
          N: 4 -> [_]
          tunnel: w4754 -> [w4783] mode=indexing
          tunnel: w4761 -> [w4784]
          tunnel: w4760 -> [w4786]
          tunnel: w4736 -> [w4779]
          tunnel: w4759 -> [w4778]
          tunnel: "# Spectra to Ave." -> [w4777]
          tunnel: [w4776] -> w4749 mode=indexing
          tunnel: w4750 -> [w4781] mode=indexing
          tunnel: [w4780] -> w4737 mode=indexing
          tunnel: w4740 -> [w4775]
          n2912 = Less?(x=w4783, y=w4786) -> (x < y?=w4785:bool)
          n2913 = Index Array(array=w4784, index=w4783) -> (element=w4782:waveform(dbl))
          n2914 = case shown="True" w4785 {
            tunnel: w4782 -> [_ w4803]
            tunnel: w4781 -> [w4788 w4801]
            tunnel: [w4788 w4789] -> w4780
            tunnel: w4779 -> [_ w4800]
            tunnel: w4778 -> [_ w4793]
            tunnel: w4777 -> [_ w4792]
            tunnel: [cluster{"f0":dbl, "df":dbl, "magnitude":dbl[]} {"f0"=0.0, "df"=0.0, "magnitude"=[]} ("PSD") w4794] -> w4776
            tunnel: w4775 -> [_ w4791]
            frame False {
            }
            frame True {
              n2915 = call <vilib>:"Std Deviation and Variance.vi"("X"=w4803) -> ("mean"=w4804:dbl)  [unwired: 1 in, 2 out]
              n2916 = Subtract(x=w4803, y=w4804) -> (x-y=w4802:waveform(dbl))
              n2917 = xnode "Spectral Measurements"("Signals"=w4802) -> ("PSD"=w4796:cluster{"f0":dbl, "df":dbl, "magnitude":dbl[]})  [unwired: 1 in, 1 out]
              n2918 = case shown="False" w4800 {
                tunnel: w4801 -> [w4813 _]
                tunnel: [w4809 w4818] -> w4789
                tunnel: w4796 -> [w4812 w4819]
                tunnel: w4793 -> [w4811 _]
                frame False {
                  n2919 = Build Array (concatenate)(w4813, w4812) -> (w4810:cluster{"f0":dbl, "df":dbl, "magnitude":dbl[]}[])
                  n2920 = case shown="True" w4811 {
                    tunnel: w4810 -> [w4814 w4817]
                    tunnel: [w4814 w4815] -> w4809
                    frame False {
                    }
                    frame True {
                      n2921 = Delete From Array(array=w4817, index=0) -> (array with subset deleted=w4815:cluster{"f0":dbl, "df":dbl, "magnitude":dbl[]}[])  [unwired: 1 in, 1 out]
                    }
                  }
                }
                frame True {
                  n2922 = Build Array(w4819) -> (w4818:cluster{"f0":dbl, "df":dbl, "magnitude":dbl[]}[])
                }
              }
              n2923 = for {
                tunnel: w4789 -> [w4808] mode=indexing
                tunnel: [w4807] -> w4799 mode=indexing
                workers-P: _ -> [_]
                n2924 = Unbundle By Name(w4808) -> ("magnitude"=w4807:dbl[])
              }
              n2925 = Transpose 2D Array(2D array=w4799) -> (transposed array=w4798:dbl[][])
              n2926 = for {
                tunnel: w4798 -> [w4806] mode=indexing
                tunnel: [w4805] -> w4797 mode=indexing
                workers-P: _ -> [_]
                n2927 = Add Array Elements(numeric array=w4806) -> (sum=w4805:dbl)
              }
              n2928 = Select(t=w4792, s=w4793, f=w4791) -> (s? t:f=w4790:dbl)
              n2929 = Divide(x=w4797, y=w4790) -> (x/y=w4795:dbl[])
              n2930 = Bundle By Name(cluster=w4796, "magnitude"=w4795) -> (w4794:cluster{"f0":dbl, "df":dbl, "magnitude":dbl[]})
            }
          }
        }
        n2931 = case shown="True" w4736 {
          tunnel: w4737 -> [w4768 w4774]
          tunnel: [w4768 w4769] -> w4735
          frame False {
          }
          frame True {
            n2932 = Array Subset(array=w4774, index (row)=0 ("index"), length (row)=4 ("length"), index (col)=0 ("index"), length (col)=1 ("length")) -> (w4769:T49)
          }
        }
        n2933 = feedback-in #23(w4735) -> ()
        n2934 = Split 1D Array(array=w4749, index=2) -> (first subarray=→"FFT 1":cluster{"f0":dbl, "df":dbl, "magnitude":dbl[]}[], second subarray=→"FFT 2":cluster{"f0":dbl, "df":dbl, "magnitude":dbl[]}[])
      }
    }
    n2935 = Index Array(array=w3452, index=4) -> (element=w3690:waveform(dbl))
    n2936 = Index Array(array=w3452, index=7) -> (element=w3687:waveform(dbl))
    n2937 = Divide(x="T1 offset_x (mV)", y=1000.0) -> (x/y=w3691:dbl)
    n2938 = feedback-in #24("Calibration") -> ()
    n2939 = feedback #24(u16 1 ("Calibration")) -> (w3709:u16)
    n2940 = Divide(x="T2 offset_x (mV)", y=1000.0) -> (x/y=w3689:dbl)
    n2941 = case shown="2" "Calibration" {
      tunnel: "T1 alpha_x (nm/V)" -> [_ w4082 w4103]
      tunnel: "T1 kappa_x (pN/nm)" -> [_ _ w4093]
      tunnel: "T2 alpha_x (nm/V)" -> [_ w4081 w4101]
      tunnel: "T2 kappa_x (pN/nm)" -> [_ _ w4094]
      tunnel: w3690 -> [w4064 w4079 w4099]
      tunnel: w3687 -> [w4063 w4077 w4097]
      tunnel: [w4064 w4076 w4096] -> w3718
      tunnel: [w4063 w4075 w4095] -> w3717
      tunnel: ["T1 X (V)" ("Label.Text") "T1 X (nm)" ("Label.Text") "T1 X (pN)" ("Label.Text")] -> w3706
      tunnel: ["T2 X (V)" ("Label.Text") "T2 X (nm)" ("Label.Text") "T2 X (pN)" ("Label.Text")] -> w3705
      tunnel: ["Position (V)" ("Label.Text") "Position (nm)" ("Label.Text") "Force (pN)" ("Label.Text")] -> w3707
      tunnel: w3689 -> [_ w4067 w4086]
      tunnel: w3691 -> [_ w4070 w4088]
      tunnel: ["Mean (V)" ("Label.Text") "Mean (nm)" ("Label.Text") "Mean (pN)" ("Label.Text")] -> w3702
      tunnel: ["Difference (V)" ("Label.Text") "Difference (nm)" ("Label.Text") "Difference (pN)" ("Label.Text")] -> w3642
      frame 0, Default {
      }
      frame 1 {
        n2942 = Unbundle By Name(w4079) -> ("Y"=w4083:dbl[])
        n2943 = Unbundle By Name(w4077) -> ("Y"=w4068:dbl[])
        n2944 = Subtract(x=w4083, y=w4070) -> (x-y=w4071:dbl[])
        n2945 = Subtract(x=w4068, y=w4067) -> (x-y=w4069:dbl[])
        n2946 = Multiply(x=w4069, y=w4081) -> (x*y=w4078:dbl[])
        n2947 = Multiply(x=w4082, y=w4071) -> (x*y=w4080:dbl[])
        n2948 = Bundle By Name(cluster=w4077, "Y"=w4078) -> (w4075:waveform(dbl))
        n2949 = Bundle By Name(cluster=w4079, "Y"=w4080) -> (w4076:waveform(dbl))
      }
      frame 2 {
        n2950 = Unbundle By Name(w4099) -> ("Y"=w4104:dbl[])
        n2951 = Unbundle By Name(w4097) -> ("Y"=w4102:dbl[])
        n2952 = Subtract(x=w4102, y=w4086) -> (x-y=w4087:dbl[])
        n2953 = Subtract(x=w4104, y=w4088) -> (x-y=w4089:dbl[])
        n2954 = Compound Arithmetic op=MULTIPLY(w4087, w4101, w4094) -> (w4098:dbl[])
        n2955 = Compound Arithmetic op=MULTIPLY(w4093, w4103, w4089) -> (w4100:dbl[])
        n2956 = Bundle By Name(cluster=w4097, "Y"=w4098) -> (w4095:waveform(dbl))
        n2957 = Bundle By Name(cluster=w4099, "Y"=w4100) -> (w4096:waveform(dbl))
      }
    }
    n2958 = case shown="True" "Read Lateness and Rel Phase" {
      tunnel: w3509 -> [w4019 w4052]
      tunnel: w3508 -> [w4020 w4051]
      tunnel: [w4019 w4024] -> w3684
      tunnel: [w4020 w4023] -> w3683
      frame False {
      }
      frame True {
        n2959 = xnode "Read/Write Control"("FPGA VI Reference In"=w4052, "error in"=w4051) -> ("FPGA VI Reference Out"=w4026:T20, "error out"=w4025:errorcluster, "GI Relative phase"=→"GI relative phase":i16, "Relative phase"=→"Relative phase (AI1)":i16, "AI Late Counter"=→"Late Counter (AI1)":u8, "GI Late Counter"=→"GI Late Counter":u8, "MCL Late Counter"=→"MCL Late Counter":u8, "MCL Relative Phase"=→"Relative Phase (MCL)":i16, "APD Acq Relative Phase"=→"APD Acq Relative Phase":i16, "APD 1 Gate Relative Phase"=→"APD 1 Gate Relative Phase":i16, "APD 2 Gate Relative Phase"=→"APD 2 Gate Relative Phase":i16, "APD Acq Late Counter"=→"APD Acq Late Counter":u8, "APD 1 Gate Late Counter"=→"APD 1 Gate Late Counter":u8, "APD 2 Gate Late Counter"=→"APD 2 Gate Late Counter":u8, "Green FB Relative Phase"=→"Relative phase (Green FB)":i16, "GI Relative phase 2"=→"GI relative phase 2":i16, "GI Late Counter 2"=→"GI Late Counter 2":u8, "Trap Pos FIFO Timeout"=→"Trap Pos FIFO Timeout":u16, "Trap AI FIFO Timeout"=→"Trap AI FIFO Timeout":u16, "RI Late Counter"=→"RI Late Counter":u8, "RI Relative phase"=→"RI relative phase":i16, "Green Late Counter"=→"Green AI Late Counter":u8, "BI Late Counter (AO)"=→"Late Counter (BI AO)":u8, "Blue Late Counter (D)"=→"Late Counter (BI DO)":u8, "BI Relative phase (AO)"=→"Relative phase (BI AO)":i16, "BI Relative phase (D)"=→"Relative phase (BI DO)":i16)